vi "真正主程序.vi"() -> ()   [LabVIEW 2013] (continued)
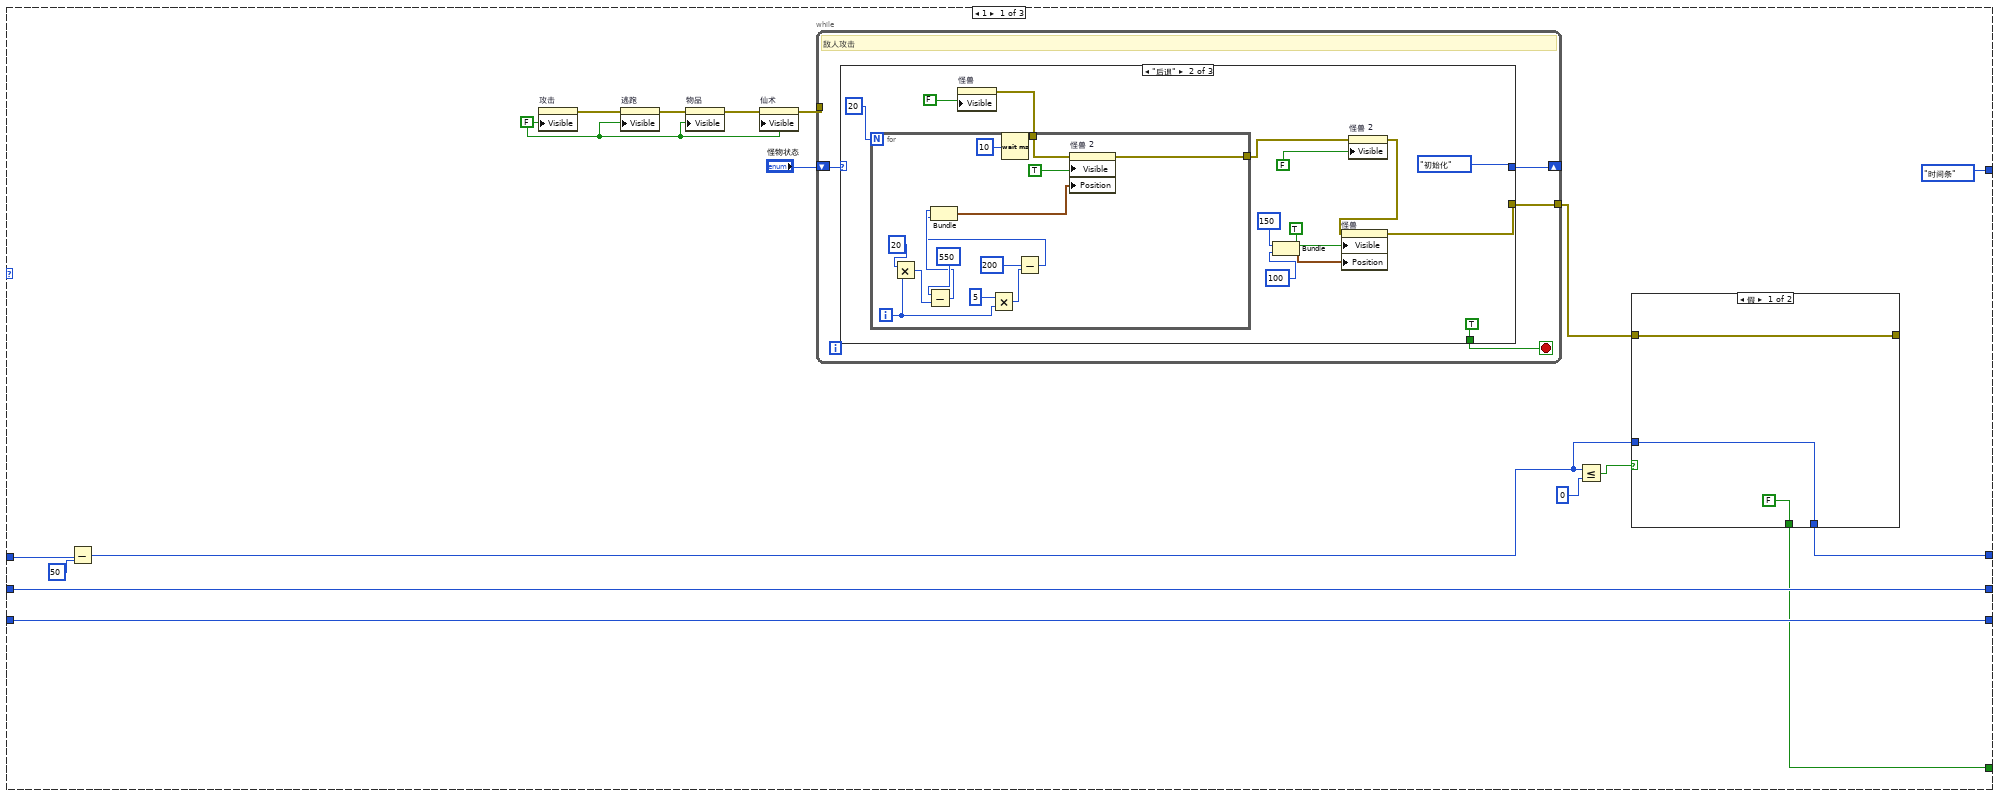
[diagram p2: hidden frame]
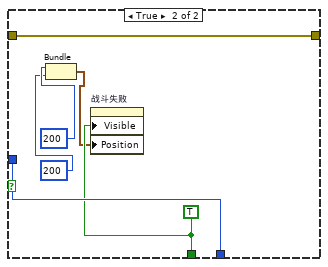
[diagram p3: hidden frame]
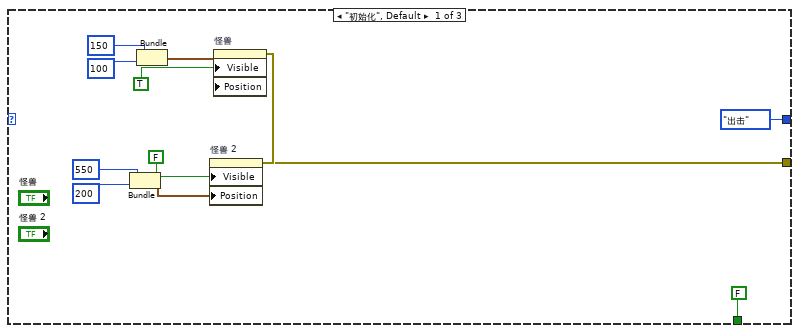
[diagram p4: hidden frame]
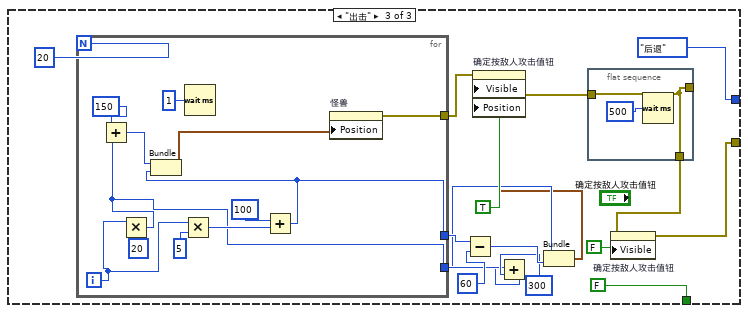
[diagram p5: hidden frame]
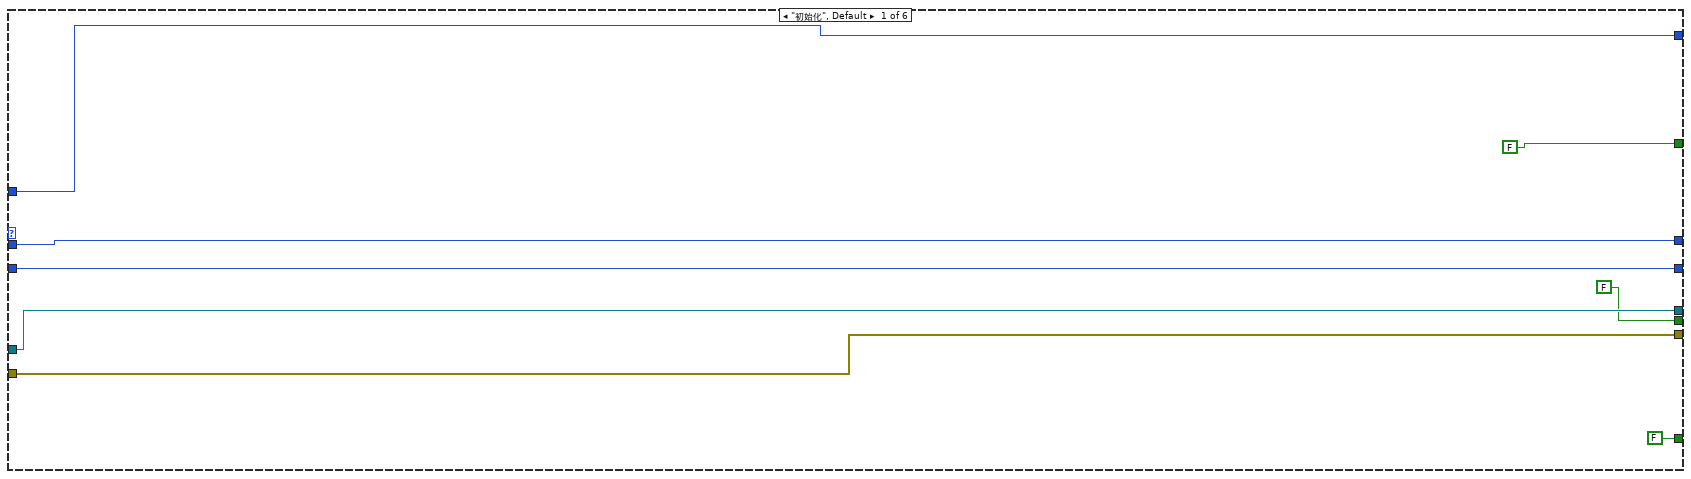
[diagram p6: hidden frame]
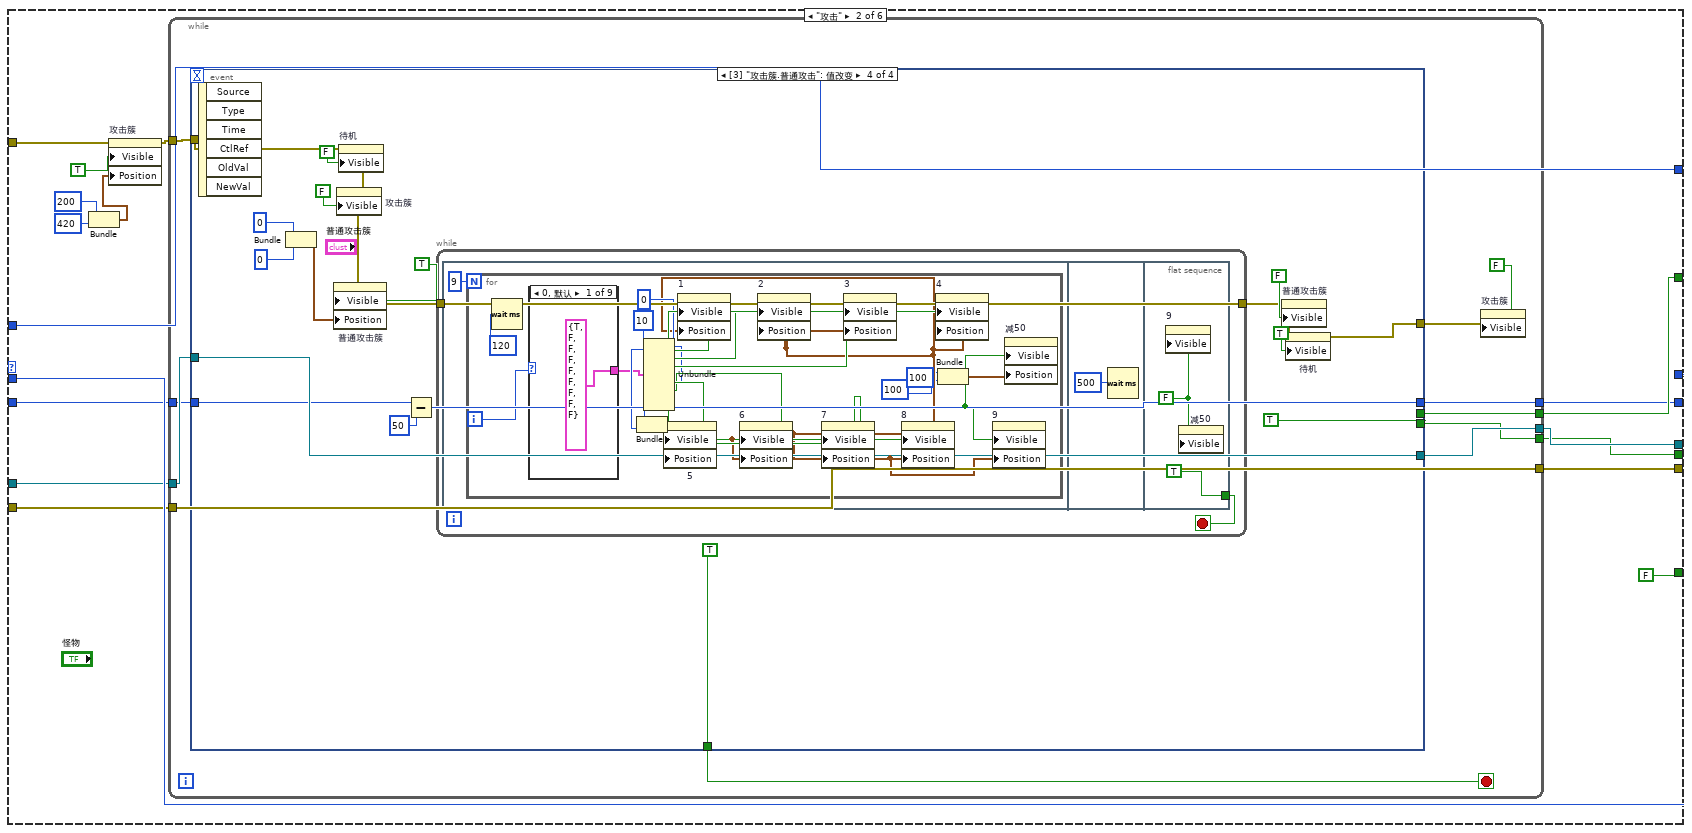
[diagram p7: hidden frame]
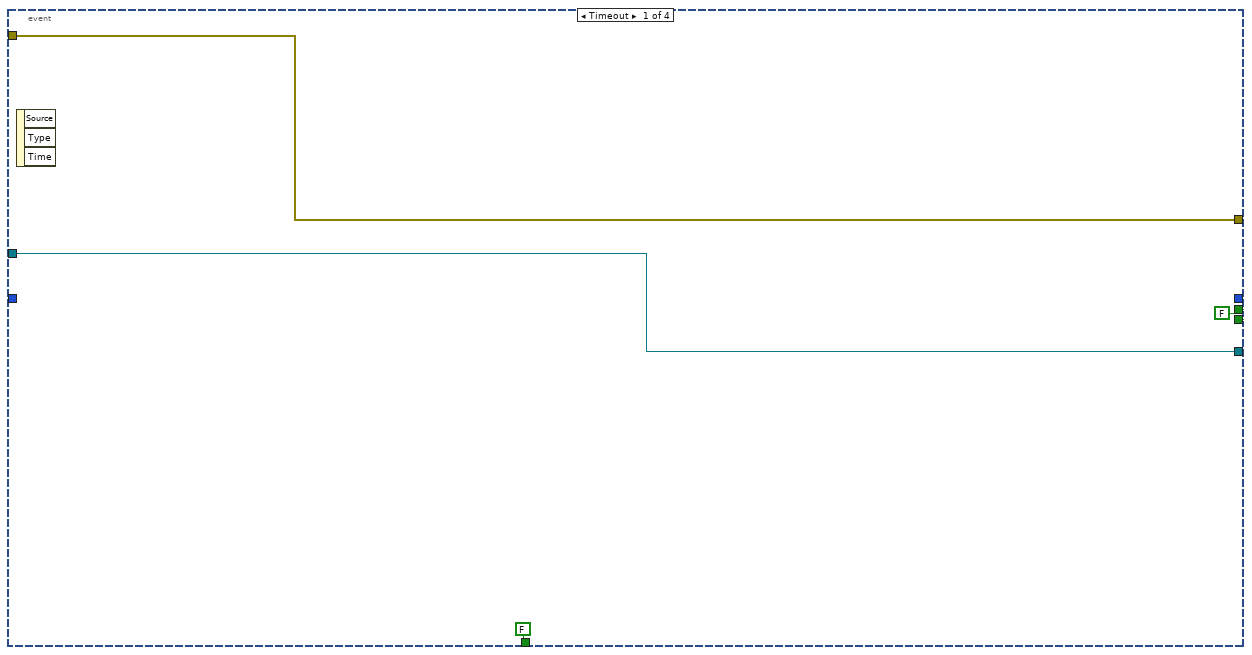
[diagram p8: hidden frame]
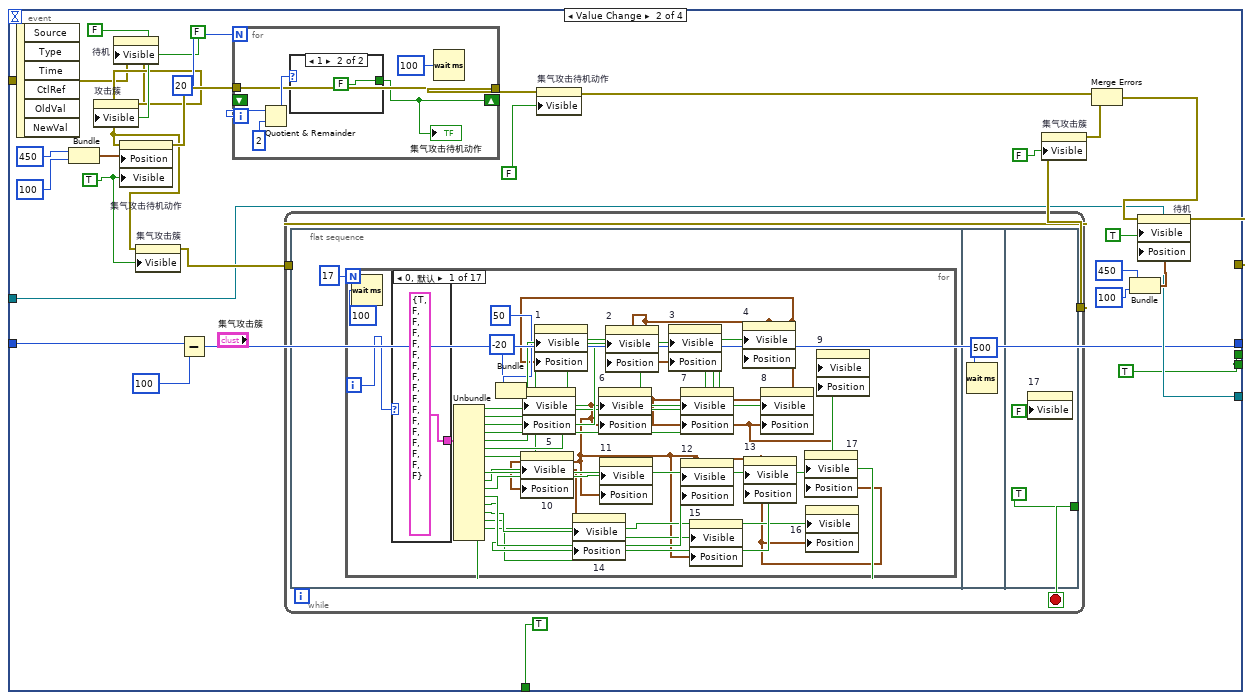
[diagram p9: hidden frame]
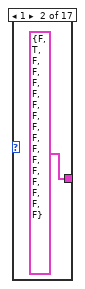
[diagram p10: hidden frame]
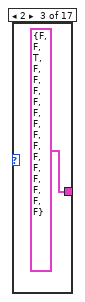
[diagram p11: hidden frame]
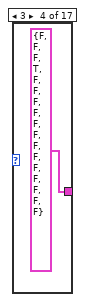
[diagram p12: hidden frame]
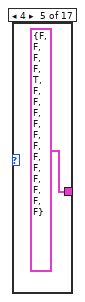
[diagram p13: hidden frame]
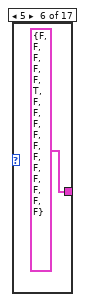
[diagram p14: hidden frame]
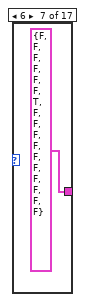
[diagram p15: hidden frame]
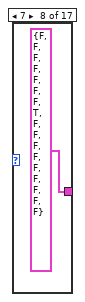
[diagram p16: hidden frame]
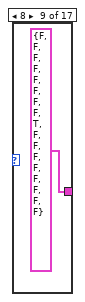
[diagram p17: hidden frame]
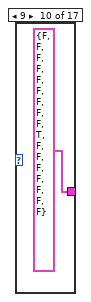
[diagram p18: hidden frame]
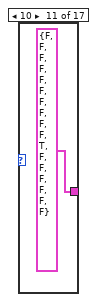
[diagram p19: hidden frame]
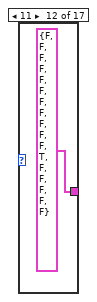
[diagram p20: hidden frame]
                                n151 = Bundle(100, 40) -> (w417:cluster{i32, i32})  [unwired: 1 in]
                                n152 = property on="10" class="Bool"("Visible"=w419, "Position"=w417) -> ()  [unwired: 2 in, 2 out]
                                n153 = property on="14" class="Bool"("Visible"=w409, "Position"=w417) -> ()  [unwired: 2 in, 2 out]
                                n154 = property on="5" class="Bool"("Visible"=w424, "Position"=w417) -> ()  [unwired: 2 in, 2 out]
                                n155 = property on="1" class="Bool"("Visible"=w428, "Position"=w417) -> ()  [unwired: 2 in, 2 out]
                                n156 = property on="6" class="Bool"("Visible"=w423, "Position"=w417) -> ()  [unwired: 2 in, 2 out]
                                n157 = property on="11" class="Bool"("Visible"=w414, "Position"=w417) -> ()  [unwired: 2 in, 2 out]
                                n158 = property on="2" class="Bool"("Visible"=w427, "Position"=w417) -> ()  [unwired: 2 in, 2 out]
                                n159 = property on="15" class="Bool"("Visible"=w406, "Position"=w417) -> ()  [unwired: 2 in, 2 out]
                                n160 = property on="7" class="Bool"("Visible"=w411, "Position"=w417) -> ()  [unwired: 2 in, 2 out]
                                n161 = property on="3" class="Bool"("Visible"=w426, "Position"=w417) -> ()  [unwired: 2 in, 2 out]
                                n162 = property on="12" class="Bool"("Visible"=w418, "Position"=w417) -> ()  [unwired: 2 in, 2 out]
                                n163 = property on="8" class="Bool"("Visible"=w410, "Position"=w417) -> ()  [unwired: 2 in, 2 out]
                                n164 = Bundle(100, 100) -> (w407:cluster{i32, i32})  [unwired: 1 in]
                                n165 = property on="4" class="Bool"("Visible"=w425, "Position"=w417) -> ()  [unwired: 2 in, 2 out]
                                n166 = property on="13" class="Bool"("Visible"=w408, "Position"=w417) -> ()  [unwired: 2 in, 2 out]
                                n167 = property on="确定按钮" class="Bool"("Visible"=w406, "Position"=w407) -> ()  [unwired: 2 in, 2 out]
                                n168 = property on="9" class="Bool"("Visible"=w420, "Position"=w417) -> ()  [unwired: 2 in, 2 out]
                              }
                            }
                            frame #1 {
                              n169 = Wait (ms)(milliseconds to wait=500) -> ()  [unwired: 1 out]
                            }
                            frame #2 {
                              n170 = property on="确定按钮" class="Bool"("Visible"=FALSE) -> ()  [unwired: 2 in, 2 out]
                              n171 = property on="15" class="Bool"("Visible"=FALSE) -> ()  [unwired: 2 in, 2 out]
                            }
                          }
                        }
                        n172 = property on="火爪术簇" class="Clust"(error in=w392, "Visible"=FALSE ("可见")) -> ()  [unwired: 1 in, 2 out]
                      }
                      event "仙术簇.凝冰术": Value Change {
                        w455 = TRUE
                        n173 = event-data() -> ()  [unwired: 1 in, 6 out]
                        n174 = Subtract(x=w453, y=50) -> (x-y=w452:i32)
                        n175 = Subtract(x=w450, y=70) -> (x-y=w449:i32)
                        n176 = Bundle(0, 0) -> (w460:cluster{i32, i32})  [unwired: 1 in]
                        n177 = property on="仙术簇" class="Clust"(error in=w463, "Visible"=FALSE) -> (error out=w466:errorcluster)  [unwired: 1 in, 1 out]
                        n178 = property on="待机" class="Bool"(error in=w466, "Visible"=TRUE) -> (error out=w464:errorcluster)  [unwired: 1 in, 1 out]
                        n179 = property on="凝冰术簇" class="Clust"(error in=w464, "Visible"=TRUE, "Position"=w460) -> (error out=w457:errorcluster)  [unwired: 1 in, 1 out]
                        n180 = while {
                          tunnel: w457 -> [w469]
                          tunnel: [w469] -> w456
                          stop <- w470 stop-if-true
                          n181 = flat-sequence {
                            tunnel: [TRUE] -> w470
                            frame #0 {
                              n182 = for {
                                N: 15 -> [_]
                                i -> [w482]
                                n183 = Wait (ms)(milliseconds to wait=100) -> ()  [unwired: 1 out]
                                n184 = case shown="14" w482 {
                                tunnel: [T3 {"4"=TRUE, "5"=FALSE, "6"=FALSE, "7"=FALSE, "8"=FALSE, "1"=FALSE, "2"=FALSE, "3"=FALSE, "9"=FALSE, "10"=FALSE, "11"=FALSE, "12"=FALSE, "13"=FALSE, "14"=FALSE, "15"=FALSE, "确定按钮"=FALSE} ("簇") T3 {"4"=FALSE, "5"=TRUE, "6"=FALSE, "7"=FALSE, "8"=FALSE, "1"=FALSE, "2"=FALSE, "3"=FALSE, "9"=FALSE, "10"=FALSE, "11"=FALSE, "12"=FALSE, "13"=FALSE, "14"=FALSE, "15"=FALSE, "确定按钮"=FALSE} ("簇") T3 {"4"=FALSE, "5"=FALSE, "6"=TRUE, "7"=FALSE, "8"=FALSE, "1"=FALSE, "2"=FALSE, "3"=FALSE, "9"=FALSE, "10"=FALSE, "11"=FALSE, "12"=FALSE, "13"=FALSE, "14"=FALSE, "15"=FALSE, "确定按钮"=FALSE} ("簇") T3 {"4"=FALSE, "5"=FALSE, "6"=FALSE, "7"=TRUE, "8"=FALSE, "1"=FALSE, "2"=FALSE, "3"=FALSE, "9"=FALSE, "10"=FALSE, "11"=FALSE, "12"=FALSE, "13"=FALSE, "14"=FALSE, "15"=FALSE, "确定按钮"=FALSE} ("簇") T3 {"4"=FALSE, "5"=FALSE, "6"=FALSE, "7"=FALSE, "8"=TRUE, "1"=FALSE, "2"=FALSE, "3"=FALSE, "9"=FALSE, "10"=FALSE, "11"=FALSE, "12"=FALSE, "13"=FALSE, "14"=FALSE, "15"=FALSE, "确定按钮"=FALSE} ("簇") T3 {"4"=FALSE, "5"=FALSE, "6"=FALSE, "7"=FALSE, "8"=FALSE, "1"=TRUE, "2"=FALSE, "3"=FALSE, "9"=FALSE, "10"=FALSE, "11"=FALSE, "12"=FALSE, "13"=FALSE, "14"=FALSE, "15"=FALSE, "确定按钮"=FALSE} ("簇") T3 {"4"=FALSE, "5"=FALSE, "6"=FALSE, "7"=FALSE, "8"=FALSE, "1"=FALSE, "2"=TRUE, "3"=FALSE, "9"=FALSE, "10"=FALSE, "11"=FALSE, "12"=FALSE, "13"=FALSE, "14"=FALSE, "15"=FALSE, "确定按钮"=FALSE} ("簇") T3 {"4"=FALSE, "5"=FALSE, "6"=FALSE, "7"=FALSE, "8"=FALSE, "1"=FALSE, "2"=FALSE, "3"=TRUE, "9"=FALSE, "10"=FALSE, "11"=FALSE, "12"=FALSE, "13"=FALSE, "14"=FALSE, "15"=FALSE, "确定按钮"=FALSE} ("簇") T3 {"4"=FALSE, "5"=FALSE, "6"=FALSE, "7"=FALSE, "8"=FALSE, "1"=FALSE, "2"=FALSE, "3"=FALSE, "9"=TRUE, "10"=FALSE, "11"=FALSE, "12"=FALSE, "13"=FALSE, "14"=FALSE, "15"=FALSE, "确定按钮"=FALSE} ("簇") T3 {"4"=FALSE, "5"=FALSE, "6"=FALSE, "7"=FALSE, "8"=FALSE, "1"=FALSE, "2"=FALSE, "3"=FALSE, "9"=FALSE, "10"=TRUE, "11"=FALSE, "12"=FALSE, "13"=FALSE, "14"=FALSE, "15"=FALSE, "确定按钮"=FALSE} ("簇") T3 {"4"=FALSE, "5"=FALSE, "6"=FALSE, "7"=FALSE, "8"=FALSE, "1"=FALSE, "2"=FALSE, "3"=FALSE, "9"=FALSE, "10"=FALSE, "11"=TRUE, "12"=FALSE, "13"=FALSE, "14"=FALSE, "15"=FALSE, "确定按钮"=FALSE} ("簇") T3 {"4"=FALSE, "5"=FALSE, "6"=FALSE, "7"=FALSE, "8"=FALSE, "1"=FALSE, "2"=FALSE, "3"=FALSE, "9"=FALSE, "10"=FALSE, "11"=FALSE, "12"=TRUE, "13"=FALSE, "14"=FALSE, "15"=FALSE, "确定按钮"=FALSE} ("簇") T3 {"4"=FALSE, "5"=FALSE, "6"=FALSE, "7"=FALSE, "8"=FALSE, "1"=FALSE, "2"=FALSE, "3"=FALSE, "9"=FALSE, "10"=FALSE, "11"=FALSE, "12"=FALSE, "13"=TRUE, "14"=FALSE, "15"=FALSE, "确定按钮"=FALSE} ("簇") T3 {"4"=FALSE, "5"=FALSE, "6"=FALSE, "7"=FALSE, "8"=FALSE, "1"=FALSE, "2"=FALSE, "3"=FALSE, "9"=FALSE, "10"=FALSE, "11"=FALSE, "12"=FALSE, "13"=FALSE, "14"=TRUE, "15"=FALSE, "确定按钮"=FALSE} ("簇") T3 {"4"=FALSE, "5"=FALSE, "6"=FALSE, "7"=FALSE, "8"=FALSE, "1"=FALSE, "2"=FALSE, "3"=FALSE, "9"=FALSE, "10"=FALSE, "11"=FALSE, "12"=FALSE, "13"=FALSE, "14"=FALSE, "15"=TRUE, "确定按钮"=FALSE} ("簇")] -> w481
                                frame 0, Default {
                                }
                                frame 1 {
                                }
                                frame 2 {
                                }
                                frame 3 {
                                }
                                frame 4 {
                                }
                                frame 5 {
                                }
                                frame 6 {
                                }
                                frame 7 {
                                }
                                frame 8 {
                                }
                                frame 9 {
                                }
                                frame 10 {
                                }
                                frame 11 {
                                }
                                frame 12 {
                                }
                                frame 13 {
                                }
                                frame 14 {
                                }
                                }
                                n185 = Unbundle(w481) -> ("4"=w494:bool, "5"=w493:bool, "6"=w492:bool, "7"=w491:bool, "8"=w490:bool, "1"=w489:bool, "2"=w477:bool, "3"=w476:bool, "9"=w486:bool, "10"=w485:bool, "11"=w480:bool, "12"=w484:bool, "13"=w474:bool, "14"=w475:bool, "15"=w472:bool)  [unwired: 1 out]
                                n186 = Bundle(150, 80) -> (w483:cluster{i32, i32})  [unwired: 1 in]
                                n187 = property on="确定按钮 10" class="Bool"("Visible"=w485, "Position"=w483) -> ()  [unwired: 2 in, 2 out]
                                n188 = property on="确定按钮 5" class="Bool"("Visible"=w490, "Position"=w483) -> ()  [unwired: 2 in, 2 out]
                                n189 = property on="确定按钮 14" class="Bool"("Visible"=w475, "Position"=w483) -> ()  [unwired: 2 in, 2 out]
                                n190 = property on="确定按钮1" class="Bool"("Visible"=w494, "Position"=w483) -> ()  [unwired: 2 in, 2 out]
                                n191 = property on="确定按钮 6" class="Bool"("Visible"=w489, "Position"=w483) -> ()  [unwired: 2 in, 2 out]
                                n192 = property on="确定按钮 11" class="Bool"("Visible"=w480, "Position"=w483) -> ()  [unwired: 2 in, 2 out]
                                n193 = property on="确定按钮 2" class="Bool"("Visible"=w493, "Position"=w483) -> ()  [unwired: 2 in, 2 out]
                                n194 = property on="确定按钮 15" class="Bool"("Visible"=w472, "Position"=w483) -> ()  [unwired: 2 in, 2 out]
                                n195 = property on="确定按钮 7" class="Bool"("Visible"=w477, "Position"=w483) -> ()  [unwired: 2 in, 2 out]
                                n196 = property on="确定按钮 3" class="Bool"("Visible"=w492, "Position"=w483) -> ()  [unwired: 2 in, 2 out]
                                n197 = property on="确定按钮 12" class="Bool"("Visible"=w484, "Position"=w483) -> ()  [unwired: 2 in, 2 out]
                                n198 = property on="确定按钮 8" class="Bool"("Visible"=w476, "Position"=w483) -> ()  [unwired: 2 in, 2 out]
                                n199 = Bundle(100, 50) -> (w473:cluster{i32, i32})  [unwired: 1 in]
                                n200 = property on="确定按钮 4" class="Bool"("Visible"=w491, "Position"=w483) -> ()  [unwired: 2 in, 2 out]
                                n201 = property on="确定按钮 13" class="Bool"("Visible"=w474, "Position"=w483) -> ()  [unwired: 2 in, 2 out]
                                n202 = property class="Bool"("Visible"=w472, "Position"=w473) -> ()  [unwired: 2 in, 2 out]
                                n203 = property on="确定按钮 9" class="Bool"("Visible"=w486, "Position"=w483) -> ()  [unwired: 2 in, 2 out]
                              }
                            }
                            frame #1 {
                              n204 = Wait (ms)(milliseconds to wait=500) -> ()  [unwired: 1 out]
                            }
                            frame #2 {
                              n205 = property on="确定按钮 15" class="Bool"("Visible"=FALSE) -> ()  [unwired: 2 in, 2 out]
                              n206 = property class="Bool"("Visible"=FALSE) -> ()  [unwired: 2 in, 2 out]
                            }
                          }
                        }
                        n207 = property on="凝冰术簇" class="Clust"(error in=w456, "Visible"=FALSE ("可见")) -> ()  [unwired: 1 in, 2 out]
                      }
                      event "仙术簇.疾风术": Value Change {
                        w521 = TRUE
                        n208 = event-data() -> ()  [unwired: 1 in, 6 out]
                        n209 = Subtract(x=w519, y=50) -> (x-y=w518:i32)
                        n210 = Bundle(0, 0) -> (w526:cluster{i32, i32})  [unwired: 1 in]
                        n211 = Subtract(x=w516, y=70) -> (x-y=w515:i32)
                        n212 = property on="仙术簇" class="Clust"(error in=w529, "Visible"=FALSE) -> (error out=w532:errorcluster)  [unwired: 1 in, 1 out]
                        n213 = property on="待机" class="Bool"(error in=w532, "Visible"=TRUE) -> (error out=w530:errorcluster)  [unwired: 1 in, 1 out]
                        n214 = property on="疾风术簇" class="Clust"(error in=w530, "Visible"=TRUE, "Position"=w526) -> (error out=w523:errorcluster)  [unwired: 1 in, 1 out]
                        n215 = while {
                          tunnel: w523 -> [w535]
                          tunnel: [w535] -> w522
                          stop <- w536 stop-if-true
                          n216 = flat-sequence {
                            tunnel: [TRUE] -> w536
                            frame #0 {
                              n217 = for {
                                N: 14 -> [_]
                                i -> [w549]
                                n218 = Wait (ms)(milliseconds to wait=100) -> ()  [unwired: 1 out]
                                n219 = case shown="13" w549 {
                                tunnel: [T3 {"4"=TRUE, "5"=FALSE, "6"=FALSE, "7"=FALSE, "8"=FALSE, "1"=FALSE, "2"=FALSE, "3"=FALSE, "9"=FALSE, "10"=FALSE, "11"=FALSE, "12"=FALSE, "13"=FALSE, "14"=FALSE, "15"=FALSE, "确定按钮"=FALSE} ("簇") T3 {"4"=FALSE, "5"=TRUE, "6"=FALSE, "7"=FALSE, "8"=FALSE, "1"=FALSE, "2"=FALSE, "3"=FALSE, "9"=FALSE, "10"=FALSE, "11"=FALSE, "12"=FALSE, "13"=FALSE, "14"=FALSE, "15"=FALSE, "确定按钮"=FALSE} ("簇") T3 {"4"=FALSE, "5"=FALSE, "6"=TRUE, "7"=FALSE, "8"=FALSE, "1"=FALSE, "2"=FALSE, "3"=FALSE, "9"=FALSE, "10"=FALSE, "11"=FALSE, "12"=FALSE, "13"=FALSE, "14"=FALSE, "15"=FALSE, "确定按钮"=FALSE} ("簇") T3 {"4"=FALSE, "5"=FALSE, "6"=FALSE, "7"=TRUE, "8"=FALSE, "1"=FALSE, "2"=FALSE, "3"=FALSE, "9"=FALSE, "10"=FALSE, "11"=FALSE, "12"=FALSE, "13"=FALSE, "14"=FALSE, "15"=FALSE, "确定按钮"=FALSE} ("簇") T3 {"4"=FALSE, "5"=FALSE, "6"=FALSE, "7"=FALSE, "8"=TRUE, "1"=FALSE, "2"=FALSE, "3"=FALSE, "9"=FALSE, "10"=FALSE, "11"=FALSE, "12"=FALSE, "13"=FALSE, "14"=FALSE, "15"=FALSE, "确定按钮"=FALSE} ("簇") T3 {"4"=FALSE, "5"=FALSE, "6"=FALSE, "7"=FALSE, "8"=FALSE, "1"=TRUE, "2"=FALSE, "3"=FALSE, "9"=FALSE, "10"=FALSE, "11"=FALSE, "12"=FALSE, "13"=FALSE, "14"=FALSE, "15"=FALSE, "确定按钮"=FALSE} ("簇") T3 {"4"=FALSE, "5"=FALSE, "6"=FALSE, "7"=FALSE, "8"=FALSE, "1"=FALSE, "2"=TRUE, "3"=FALSE, "9"=FALSE, "10"=FALSE, "11"=FALSE, "12"=FALSE, "13"=FALSE, "14"=FALSE, "15"=FALSE, "确定按钮"=FALSE} ("簇") T3 {"4"=FALSE, "5"=FALSE, "6"=FALSE, "7"=FALSE, "8"=FALSE, "1"=FALSE, "2"=FALSE, "3"=TRUE, "9"=FALSE, "10"=FALSE, "11"=FALSE, "12"=FALSE, "13"=FALSE, "14"=FALSE, "15"=FALSE, "确定按钮"=FALSE} ("簇") T3 {"4"=FALSE, "5"=FALSE, "6"=FALSE, "7"=FALSE, "8"=FALSE, "1"=FALSE, "2"=FALSE, "3"=FALSE, "9"=TRUE, "10"=FALSE, "11"=FALSE, "12"=FALSE, "13"=FALSE, "14"=FALSE, "15"=FALSE, "确定按钮"=FALSE} ("簇") T3 {"4"=FALSE, "5"=FALSE, "6"=FALSE, "7"=FALSE, "8"=FALSE, "1"=FALSE, "2"=FALSE, "3"=FALSE, "9"=FALSE, "10"=TRUE, "11"=FALSE, "12"=FALSE, "13"=FALSE, "14"=FALSE, "15"=FALSE, "确定按钮"=FALSE} ("簇") T3 {"4"=FALSE, "5"=FALSE, "6"=FALSE, "7"=FALSE, "8"=FALSE, "1"=FALSE, "2"=FALSE, "3"=FALSE, "9"=FALSE, "10"=FALSE, "11"=TRUE, "12"=FALSE, "13"=FALSE, "14"=FALSE, "15"=FALSE, "确定按钮"=FALSE} ("簇") T3 {"4"=FALSE, "5"=FALSE, "6"=FALSE, "7"=FALSE, "8"=FALSE, "1"=FALSE, "2"=FALSE, "3"=FALSE, "9"=FALSE, "10"=FALSE, "11"=FALSE, "12"=TRUE, "13"=FALSE, "14"=FALSE, "15"=FALSE, "确定按钮"=FALSE} ("簇") T3 {"4"=FALSE, "5"=FALSE, "6"=FALSE, "7"=FALSE, "8"=FALSE, "1"=FALSE, "2"=FALSE, "3"=FALSE, "9"=FALSE, "10"=FALSE, "11"=FALSE, "12"=FALSE, "13"=TRUE, "14"=FALSE, "15"=FALSE, "确定按钮"=FALSE} ("簇") T3 {"4"=FALSE, "5"=FALSE, "6"=FALSE, "7"=FALSE, "8"=FALSE, "1"=FALSE, "2"=FALSE, "3"=FALSE, "9"=FALSE, "10"=FALSE, "11"=FALSE, "12"=FALSE, "13"=FALSE, "14"=TRUE, "15"=FALSE, "确定按钮"=FALSE} ("簇")] -> w548
                                frame 0, Default {
                                }
                                frame 1 {
                                }
                                frame 2 {
                                }
                                frame 3 {
                                }
                                frame 4 {
                                }
                                frame 5 {
                                }
                                frame 6 {
                                }
                                frame 7 {
                                }
                                frame 8 {
                                }
                                frame 9 {
                                }
                                frame 10 {
                                }
                                frame 11 {
                                }
                                frame 12 {
                                }
                                frame 13 {
                                }
                                }
                                n220 = Unbundle(w548) -> ("4"=w560:bool, "5"=w559:bool, "6"=w558:bool, "7"=w557:bool, "8"=w556:bool, "1"=w555:bool, "2"=w545:bool, "3"=w544:bool, "9"=w552:bool, "10"=w551:bool, "11"=w542:bool, "12"=w541:bool, "13"=w540:bool, "14"=w539:bool)  [unwired: 2 out]
                                n221 = Bundle(150, 50) -> (w550:cluster{i32, i32})  [unwired: 1 in]
                                n222 = property on="确定按钮 10" class="Bool"("Visible"=w551, "Position"=w550) -> ()  [unwired: 2 in, 2 out]
                                n223 = property on="确定按钮 5" class="Bool"("Visible"=w556, "Position"=w550) -> ()  [unwired: 2 in, 2 out]
                                n224 = property on="确定按钮 14" class="Bool"("Visible"=w539, "Position"=w550) -> ()  [unwired: 2 in, 2 out]
                                n225 = property on="确定按钮" class="Bool"("Visible"=w560, "Position"=w550) -> ()  [unwired: 2 in, 2 out]
                                n226 = property on="确定按钮 6" class="Bool"("Visible"=w555, "Position"=w550) -> ()  [unwired: 2 in, 2 out]
                                n227 = property on="确定按钮 11" class="Bool"("Visible"=w542, "Position"=w550) -> ()  [unwired: 2 in, 2 out]
                                n228 = property on="确定按钮 2" class="Bool"("Visible"=w559, "Position"=w550) -> ()  [unwired: 2 in, 2 out]
                                n229 = Compound Arithmetic op=OR(w542, w541, w540, w539) -> (w538:bool)
                                n230 = property on="确定按钮 7" class="Bool"("Visible"=w545, "Position"=w550) -> ()  [unwired: 2 in, 2 out]
                                n231 = property on="确定按钮 3" class="Bool"("Visible"=w558, "Position"=w550) -> ()  [unwired: 2 in, 2 out]
                                n232 = property on="确定按钮 12" class="Bool"("Visible"=w541, "Position"=w550) -> ()  [unwired: 2 in, 2 out]
                                n233 = property on="确定按钮 8" class="Bool"("Visible"=w544, "Position"=w550) -> ()  [unwired: 2 in, 2 out]
                                n234 = Bundle(150, 80) -> (w543:cluster{i32, i32})  [unwired: 1 in]
                                n235 = property on="确定按钮 4" class="Bool"("Visible"=w557, "Position"=w550) -> ()  [unwired: 2 in, 2 out]
                                n236 = property on="确定按钮 13" class="Bool"("Visible"=w540, "Position"=w550) -> ()  [unwired: 2 in, 2 out]
                                n237 = property on="确定按钮 15" class="Bool"("Visible"=w538, "Position"=w543) -> ()  [unwired: 2 in, 2 out]
                                n238 = property on="确定按钮 9" class="Bool"("Visible"=w552, "Position"=w550) -> ()  [unwired: 2 in, 2 out]
                              }
                            }
                            frame #1 {
                              n239 = Wait (ms)(milliseconds to wait=500) -> ()  [unwired: 1 out]
                            }
                            frame #2 {
                              n240 = property on="确定按钮 14" class="Bool"("Visible"=FALSE) -> ()  [unwired: 2 in, 2 out]
                              n241 = property on="确定按钮 15" class="Bool"("Visible"=FALSE) -> ()  [unwired: 2 in, 2 out]
                            }
                          }
                        }
                        n242 = property on="疾风术簇" class="Clust"(error in=w522, "Visible"=FALSE ("可见")) -> ()  [unwired: 1 in, 2 out]
                      }
                      event "仙术簇.仙术中的放弃": Value Change {
                        w582 = FALSE
                        n243 = event-data() -> ()  [unwired: 1 in, 6 out]
                        n244 = property on="仙术簇" class="Clust"(error in=w583, "Visible"=FALSE) -> ()  [unwired: 1 in, 2 out]
                      }
                    }
                  }
                }
                frame "物品" {
                  w592 = FALSE
                  n245 = Bundle(200, 420) -> (w601:cluster{i32, i32})  [unwired: 1 in]
                  n246 = property on="物品簇" class="Clust"(error in=w605, "Visible"=TRUE, "Position"=w601) -> (error out=w604:errorcluster)  [unwired: 1 in, 1 out]
                  n247 = while {
                    tunnel: w604 -> [w613]
                    tunnel: w600 -> [w612]
                    tunnel: [w609] -> w599
                    tunnel: [w611] -> w595
                    tunnel: w594 -> [w610]
                    tunnel: [w608] -> w593
                    tunnel: [w607] -> w588
                    stop <- w614 stop-if-true
                    n248 = event shown="[4] \"物品簇.鼠儿果\": 值改变" {
                      selector: _ -> [_ _ _ _ _ _]
                      dyn-events: _ -> [_ _ _ _ _ _]
                      timeout: _ -> [_ _ _ _ _ _]
                      tunnel: [w618 _ w633 w649 w663 w675] -> w611
                      tunnel: [FALSE FALSE FALSE TRUE TRUE TRUE] -> w614
                      tunnel: w613 -> [w618 w629 w643 w649 w663 w675]
                      tunnel: w612 -> [w617 w624 w638 w650 w661 w674]
                      tunnel: [w617 w624 w638 w651 w661 w674] -> w609
                      tunnel: w610 -> [w616 w623 w637 w648 w662 w672]
                      tunnel: [w616 w623 w637 w648 w660 w672] -> w608
                      tunnel: [FALSE w620 w635 TRUE TRUE FALSE] -> w607
                      event Timeout {
                        n249 = event-data() -> ()  [unwired: 1 in, 3 out]
                      }
                      event "物品簇.止血草": Mouse Enter {
                        w620 = FALSE
                        (unwired) 10
                        n250 = event-data() -> ()  [unwired: 1 in, 4 out]
                        n251 = Bundle(400, 200) -> (w625:cluster{i32, i32})  [unwired: 1 in]
                        n252 = property on="琉璃法珠簇" class="Clust"(error in=w629, "Visible"=TRUE, "Position"=w625) -> (error out=w622:errorcluster)  [unwired: 1 in, 1 out]
                        n253 = flat-sequence {
                          tunnel: w622 -> [w631]
                          tunnel: [w631] -> w621
                          frame #0 {
                            n254 = Wait (ms)(milliseconds to wait=1000) -> ()  [unwired: 1 out]
                          }
                        }
                        n255 = property on="琉璃法珠簇" class="Clust"(error in=w621, "Visible"=w620) -> ()  [unwired: 1 in, 2 out]
                      }
                      event "物品簇.鼠儿果": Mouse Enter {
                        w635 = FALSE
                        (unwired) 10
                        n256 = event-data() -> ()  [unwired: 1 in, 4 out]
                        n257 = Bundle(400, 200) -> (w639:cluster{i32, i32})  [unwired: 1 in]
                        n258 = property on="龙蟠雕玉" class="Clust"(error in=w643, "Visible"=TRUE, "Position"=w639) -> (error out=w636:errorcluster)  [unwired: 1 in, 1 out]
                        n259 = flat-sequence {
                          tunnel: w636 -> [w645]
                          tunnel: [w645] -> w634
                          frame #0 {
                            n260 = Wait (ms)(milliseconds to wait=1000) -> ()  [unwired: 1 out]
                          }
                        }
                        n261 = property on="龙蟠雕玉" class="Clust"(error in=w634, "Visible"=w635) -> (error out=w633:errorcluster)  [unwired: 1 in, 1 out]
                      }
                      event "物品簇.止血草": Value Change {
                        n262 = event-data() -> ()  [unwired: 1 in, 6 out]
                        n263 = Greater?(x=w650, y=100) -> (0:w652:bool)
                        n264 = case shown="真" w652 {
                          tunnel: [w655 200] -> w651
                          tunnel: w650 -> [w657 _]
                          frame False {
                            n265 = Add(x=w657, y=100) -> (x+y=w655:i32)
                          }
                          frame True {
                          }
                        }
                      }
                      event "物品簇.鼠儿果": Value Change {
                        n266 = event-data() -> ()  [unwired: 1 in, 6 out]
                        n267 = Greater?(x=w662, y=150) -> (0:w664:bool)
                        n268 = case shown="假" w664 {
                          tunnel: [w668 200] -> w660
                          tunnel: w662 -> [w667 _]
                          frame False {
                            n269 = Add(x=w667, y=50) -> (x+y=w668:i32)
                          }
                          frame True {
                          }
                        }
                      }
                      event "物品簇.物品中的放弃": Value Change {
                        n270 = event-data() -> ()  [unwired: 1 in, 6 out]
                      }
                    }
                  }
                  n271 = Bundle(200, 420) -> (w596:cluster{i32, i32})  [unwired: 1 in]
                  n272 = property on="物品簇" class="Clust"(error in=w595, "Visible"=w592, "Position"=w596) -> (error out=w591:errorcluster)  [unwired: 1 in, 1 out]
                  n273 = property on="龙蟠雕玉" class="Clust"(error in=w591, "Visible"=w592) -> ()  [unwired: 1 in, 2 out]
                  n274 = property on="琉璃法珠簇" class="Clust"(error in=w591, "Visible"=w592) -> ()  [unwired: 1 in, 2 out]
                }
                frame "逃跑" {
                  n275 = Bundle(200, 140) -> (w685:cluster{i32, i32})  [unwired: 1 in]
                  n276 = property on="逃跑成功" class="Bool"(error in=w690, "Visible"=TRUE, "Position"=w685) -> (error out=w684:errorcluster)  [unwired: 1 in, 1 out]
                  n277 = flat-sequence {
                    tunnel: w684 -> [w692]
                    tunnel: [TRUE] -> w683
                    tunnel: [w692] -> w677
                    frame #0 {
                      n278 = Wait (ms)(milliseconds to wait=1500) -> ()  [unwired: 1 out]
                    }
                  }
                  n279 = property on="逃跑成功" class="Bool"(error in=w677, "Visible"=FALSE) -> ()  [unwired: 1 in, 2 out]
                }
                frame "神不足" {
                  n280 = Bundle(400, 400) -> (w697:cluster{i32, i32})  [unwired: 1 in]
                  n281 = property on="神值不够" class="Bool"("Visible"=FALSE, "Position"=w697) -> (error out=w701:errorcluster)  [unwired: 2 in, 1 out]
                  n282 = flat-sequence {
                    tunnel: w701 -> [w711]
                    tunnel: [w710] -> w700
                    frame #0 {
                      n283 = property on="神值不够" class="Bool"(error in=w711, "Visible"=TRUE) -> (error out=w710:errorcluster)  [unwired: 1 in, 1 out]
                      n284 = Wait (ms)(milliseconds to wait=2000) -> ()  [unwired: 1 out]
                    }
                  }
                  n285 = property on="神值不够" class="Bool"(error in=w700, "Visible"=FALSE) -> ()  [unwired: 1 in, 2 out]
                }
              }
              n286 = Send Notification(notification=w160, notifier=w161, error in (no error)=w159) -> (notifier out=w157:refnum<notifier>, error out=w158:errorcluster)
              n287 = Or(x=w166, y=FALSE) -> (x .or. y?=w164:bool)
              "五个状态 2" <- w156
            }
            frame Error {
            }
          }
        }
        n288 = while {
          tunnel: w134 -> [w728]
          tunnel: w127 -> [w726]
          tunnel: w122 -> [_]
          shift-right: [w721] -> w116
          shift-left: w135 -> [w727]
          stop <- w722 stop-if-true
          n289 = Wait on Notification(notifier=w726) -> (notification=w725:bool)  [unwired: 3 in, 3 out]
          n290 = Bundle(450, 100) -> (w735:cluster{i32, i32})  [unwired: 1 in]
          n291 = property on="待机" class="Bool"(error in=w727, "Visible"=TRUE, "Position"=w735) -> (error out=w734:errorcluster)  [unwired: 1 in, 1 out]
          n292 = property on="逃跑成功" class="Bool"(error in=w734, "Visible"=FALSE ("可见")) -> (error out=w733:errorcluster)  [unwired: 1 in, 1 out]
          n293 = event shown="[3] \"仙术\": 值改变" {
            selector: _ -> [_ _ _ _]
            dyn-events: _ -> [_ _ _ _]
            timeout: _ -> [_ _ _ _]
            tunnel: w728 -> [w752 w761 w768 w778]
            tunnel: w733 -> [w751 w760 w767 w777]
            tunnel: [w747 w759 w766 w776] -> w721
            tunnel: [cluster{bool, bool, bool, bool} {TRUE, FALSE, FALSE, FALSE} cluster{bool, bool, bool, bool} {FALSE, FALSE, FALSE, FALSE} cluster{bool, bool, bool, bool} {FALSE, TRUE, FALSE, FALSE} w769] -> w743
            tunnel: [FALSE TRUE FALSE FALSE] -> w723
            event "攻击": Value Change {
              n294 = event-data() -> ()  [unwired: 1 in, 2 out]
              n295 = Enqueue Element(queue=w752, element=enum16{"神不足", "逃跑", "初始化", "物品", "仙术", "攻击"}."攻击" ("五个状态"), error in (no error)=w751) -> (error out=w745:errorcluster)  [unwired: 1 in, 2 out]
              n296 = property on="集气攻击待机动作" class="Bool"(error in=w745, "Visible"=FALSE) -> (error out=w748:errorcluster)  [unwired: 1 in, 1 out]
              n297 = invoke on="攻击" class="Bool" method="Reinit To Default"(error in=w748) -> (error out=w747:errorcluster)  [unwired: 2 in, 2 out]
            }
            event "逃跑": Value Change {
              n298 = event-data() -> ()  [unwired: 1 in, 2 out]
              n299 = Enqueue Element(queue=w761, element=enum16{"神不足", "逃跑", "初始化", "物品", "仙术", "攻击"}."逃跑" ("五个状态"), error in (no error)=w760) -> (error out=w756:errorcluster)  [unwired: 1 in, 2 out]
              n300 = property on="集气攻击待机动作" class="Bool"(error in=w756, "Visible"=FALSE) -> (error out=w758:errorcluster)  [unwired: 1 in, 1 out]
              n301 = invoke on="逃跑" class="Bool" method="Reinit To Default"(error in=w758) -> (error out=w759:errorcluster)  [unwired: 2 in, 2 out]
            }
            event "物品": Value Change {
              n302 = event-data() -> ()  [unwired: 1 in, 2 out]
              n303 = Enqueue Element(queue=w768, element=enum16{"神不足", "逃跑", "初始化", "物品", "仙术", "攻击"}."物品" ("五个状态"), error in (no error)=w767) -> (error out=w765:errorcluster)  [unwired: 1 in, 2 out]
              n304 = invoke on="物品" class="Bool" method="Reinit To Default"(error in=w765) -> (error out=w766:errorcluster)  [unwired: 2 in, 2 out]
            }
            event "仙术": Value Change {
              n305 = event-data() -> ()  [unwired: 1 in, 2 out]
              n306 = property on="神" class="Slide (严格)"() -> ("Value"=w772:i32)  [unwired: 2 in, 2 out]
              n307 = Less Or Equal?(x=w772, y=0) -> (x <= y?=w773:bool)
              n308 = case shown="假" w773 {
                tunnel: [enum16{"神不足", "逃跑", "初始化", "物品", "仙术", "攻击"}."仙术" ("五个状态") enum16{"神不足", "逃跑", "初始化", "物品", "仙术", "攻击"}."神不足" ("五个状态")] -> w770
                tunnel: [cluster{bool, bool, bool, bool} {FALSE, FALSE, TRUE, FALSE} cluster{bool, bool, bool, bool} {FALSE, FALSE, FALSE, FALSE}] -> w769
                frame False {
                }
                frame True {
                }
              }
              n309 = Enqueue Element(queue=w778, element=w770, error in (no error)=w777) -> (error out=w775:errorcluster)  [unwired: 1 in, 2 out]
              n310 = invoke on="仙术" class="Bool" method="Reinit To Default"(error in=w775) -> (error out=w776:errorcluster)  [unwired: 2 in, 2 out]
            }
          }
          n311 = Unbundle(w743) -> (w742:bool, w741:bool, w740:bool, w739:bool)
          n312 = property on="琉璃法珠簇" class="Clust"("Visible"=w739) -> ()  [unwired: 2 in, 2 out]
          n313 = property on="集气攻击簇" class="Clust"("Visible"=w739) -> ()  [unwired: 2 in, 2 out]
          n314 = Unbundle By Name(w721) -> ("status"=w724:bool)
          n315 = Compound Arithmetic op=OR(w725, w724, w723) -> (w722:bool)
          n316 = Bundle(200, 420) -> (w729:cluster{i32, i32})  [unwired: 1 in]
          n317 = property on="物品簇" class="Clust"("Visible"=w741, "Position"=w729) -> ()  [unwired: 2 in, 2 out]
          n318 = property on="仙术簇" class="Clust"("Visible"=w740, "Position"=w729) -> ()  [unwired: 2 in, 2 out]
          n319 = property on="攻击簇" class="Clust"("Visible"=w742, "Position"=w729) -> ()  [unwired: 2 in, 2 out]
        }
        n320 = Release Queue(queue=w134, error in (no error)=w116) -> (error out=w133:errorcluster)  [unwired: 1 in, 2 out]
        n321 = flat-sequence {
          tunnel: w133 -> [w137]
          tunnel: [w137] -> _
          tunnel: [enum16{"我方攻击", "敌人战斗", "时间条"}."时间条" ("枚举")] -> w132
          frame #0 {
          }
        }
        n322 = Release Notifier(notifier=w130, error in (no error)=w129) -> ()  [unwired: 1 in, 3 out]
      }
      frame 2, Default {
        w783 = FALSE
        n323 = Greater Or Equal?(x=w786, y=0) -> (x >= y?=w787:bool)
        n324 = property on="战斗胜利" class="Bool"("Visible"=w783) -> ()  [unwired: 2 in, 2 out]
        n325 = property on="战斗失败" class="Bool"("Visible"=w783) -> ()  [unwired: 2 in, 2 out]
        n326 = case shown="真" w787 {
          tunnel: [enum16{"我方攻击", "敌人战斗", "时间条"}."敌人战斗" ("枚举") w803] -> w790
          tunnel: [TRUE FALSE] -> w785
          frame False {
            n327 = Bundle(200, 200) -> (w791:cluster{i32, i32})  [unwired: 1 in]
            n328 = property on="战斗胜利" class="Bool"("Visible"=TRUE, "Position"=w791) -> ()  [unwired: 2 in, 2 out]
          }
          frame True {
            w799 = FALSE
            n329 = property on="物品" class="Bool"("Visible"=w799) -> (error out=w802:errorcluster)  [unwired: 2 in, 1 out]
            n330 = property on="逃跑" class="Bool"(error in=w802, "Visible"=w799) -> (error out=w801:errorcluster)  [unwired: 1 in, 1 out]
            n331 = property on="仙术" class="Bool"(error in=w801, "Visible"=w799) -> (error out=w800:errorcluster)  [unwired: 1 in, 1 out]
            n332 = property on="攻击" class="Bool"(error in=w800, "Visible"=w799) -> (error out=w798:errorcluster)  [unwired: 1 in, 1 out]
            n333 = while {
              shift-right: [w809] -> _
              shift-left: _ -> [w818]
              shift-right: [w810] -> _
              shift-left: _ -> [w819]
              tunnel: 4 -> [w820]
              tunnel: [w812] -> w803
              tunnel: 5 -> [w808]
              tunnel: w798 -> [_]
              stop <- w815 stop-if-true
              # "时间条进程"
              n334 = Add(x=w818, y=w808) -> (x+y=w806:i32)
              "人物行走" <- w806
              n335 = Add(x=w819, y=w820) -> (x+y=w807:i32)
              "怪物行走" <- w807
              n336 = Wait (ms)(milliseconds to wait=100) -> ()  [unwired: 1 out]
              n337 = Greater?(x=w806, y=100) -> (0:w813:bool)
              n338 = Greater?(x=w807, y=100) -> (0:w814:bool)
              n339 = Or(x=w814, y=w813) -> (x .or. y?=w815:bool)
              n340 = case shown="假" w814 {
                tunnel: [enum16{"我方攻击", "敌人战斗", "时间条"}."敌人战斗" ("枚举") w828] -> w812
                tunnel: w813 -> [_ w827]
                tunnel: [0 w826] -> w810
                tunnel: w807 -> [_ w826]
                tunnel: [w822 w825] -> w809
                tunnel: w806 -> [w822 w824]
                frame True {
                }
                frame False {
                  n341 = case shown="真" w827 {
                    tunnel: [enum16{"我方攻击", "敌方攻击", "时间条", ""}."时间条" ("主控") enum16{"我方攻击", "敌方攻击", "时间条", ""}."我方攻击" ("主控")] -> w828
                    tunnel: [w830 0] -> w825
                    tunnel: w824 -> [w830 _]
                    frame False {
                    }
                    frame True {
                    }
                  }
                }
              }
            }
          }
        }
      }
    }
    "神" <- w9
    "沈欺霜" <- w8
    "怪物血值" <- w5
  }
